vi "UHR-Fleezers Control (host) - 12.8.1.vi"() -> ()   [LabVIEW 2012] (continued)
          tunnel: [w4493 w4495] -> w4446
          tunnel: [w4492 w4494] -> w4445
          tunnel: w4448 -> [w4493 w4498]
          tunnel: w4447 -> [w4492 w4497]
          frame False {
          }
          frame True {
            n2536 = call "reset FPGA DMA.vi"("error in"=w4497, "FPGA VI Reference In"=w4498) -> ("error out"=w4494:errorcluster, "FPGA VI Reference Out"=w4495:T24)
            n2537 = local write "Overflow (data lost)"(FALSE ("Overflow (data lost)")) -> ()
          }
        }
        n2538 = case shown="False" w4436 {
          selector: w4436 -> [_ w4452]
          tunnel: w4435 -> [w4451 _]
          tunnel: [w4451 w4452] -> w4434
          frame False {
            n2539 = property on="2D or 1D Scan" class="Bool (strict)"("Val(Sgnl)"=w4451) -> ()  [unwired: 2 in, 2 out]
            n2540 = property on="Confocal Image" class="Bool (strict)"("Value"=FALSE ("Start Confocal Map")) -> ()  [unwired: 2 in, 2 out]
          }
          frame True {
          }
        }
        n2541 = local write "MCL Scanning"(w4441) -> ()
        n2542 = local read "AO1"() -> (w4438:dbl)
        n2543 = local read "AO2"() -> (w4437:dbl)
        n2544 = case shown="True" "Center Scan" {
          tunnel: w4446 -> [w4459 w4491]
          tunnel: w4445 -> [w4458 w4490]
          tunnel: [w4457 w4489] -> w4443
          tunnel: [w4456 w4488] -> w4442
          tunnel: [w4454 w4475] -> w4440
          tunnel: [w4453 w4474] -> w4439
          tunnel: w4438 -> [w4454 w4480]
          tunnel: w4437 -> [w4453 w4483]
          tunnel: w4434 -> [_ _]
          frame False {
            w4455 = TRUE ("AI to FIFO")
            n2545 = xnode "Read/Write Control"("FPGA VI Reference In"=w4459, "error in"=w4458, "AI to FIFO"=w4455, "APD to FIFO"=w4455, "Start scan (MCL)"=w4455) -> ("FPGA VI Reference Out"=w4457:T24, "error out"=w4456:errorcluster)
          }
          frame True {
            w4487 = TRUE ("AI to FIFO")
            n2546 = local read "Scan steps (MCL)"() -> (w4466:u64)
            n2547 = local read "Scan lines (y)"() -> (w4462:u64)
            n2548 = local read "Fast Scan Dir"() -> (w4473:bool)
            n2549 = local read "Actual MCL Inc (V)"() -> (w4463:dbl)
            n2550 = Decrement(x=w4462) -> (x-1=w4461:u64)
            n2551 = Decrement(x=w4466) -> (x-1=w4465:u64)
            n2552 = Multiply(x=w4463, y=w4461) -> (x*y=w4460:dbl)
            n2553 = Divide(x=w4460, y=2.0) -> (x/y=w4470:dbl)
            n2554 = Multiply(x=w4463, y=w4465) -> (x*y=w4464:dbl)
            n2555 = Divide(x=w4464, y=2.0) -> (x/y=w4469:dbl)
            n2556 = Select(t=w4469, s=w4473, f=w4470) -> (s? t:f=w4468:dbl)
            n2557 = Select(t=w4470, s=w4473, f=w4469) -> (s? t:f=w4472:dbl)
            n2558 = Subtract(x=w4480, y=w4472) -> (x-y=w4471:dbl)
            n2559 = Subtract(x=w4483, y=w4468) -> (x-y=w4467:dbl)
            n2560 = local read "2D or 1D Scan"() -> (w4485:bool)
            n2561 = Not(x=w4473) -> (.not. x?=w4479:bool)
            n2562 = Not(x=w4485) -> (.not. x?=w4481:bool)
            n2563 = And(x=w4473, y=w4481) -> (x .and. y?=w4482:bool)
            n2564 = And(x=w4481, y=w4479) -> (x .and. y?=w4484:bool)
            n2565 = Select(t=w4483, s=w4484, f=w4467) -> (s? t:f=w4474:dbl)
            n2566 = Select(t=w4480, s=w4482, f=w4471) -> (s? t:f=w4475:dbl)
            n2567 = call "Volt to I16.vi"("Voltage In"=w4475) -> ("I16 Voltage Out"=w4478:i16)
            n2568 = call "Volt to I16.vi"("Voltage In"=w4474) -> ("I16 Voltage Out"=w4477:i16)
            n2569 = xnode "Read/Write Control"("FPGA VI Reference In"=w4491, "error in"=w4490, "AI to FIFO"=w4487, "APD to FIFO"=w4487, "Start scan (MCL)"=w4487, "AO1"=w4478, "AO2"=w4477) -> ("FPGA VI Reference Out"=w4489:T24, "error out"=w4488:errorcluster)
          }
        }
        "Initial Y" <- w4440
        "Initial X" <- w4439
        n2570 = local write "Tab Control 6"(T3."Imaging" ("Tab Control 6")) -> ()
        "wait to reset values" <- w4441
      }
    }
    n2571 = local read "APD Elements/DMA read"() -> (w3617:u32)
    n2572 = local read "Trap AI Elements/DMA read"() -> (w3824:u32)
    n2573 = xnode "Get APD Data"("FPGA VI Reference In"=w3770, "error in"=w3769, "Number of Elements"=w3617, "Timeout (ms)"=-1) -> ("Data"=w3798:u32[], "Elements Remaining"=→"APD FIFO Elements Remaining":u32)  [unwired: 2 out]
    n2574 = local read "Trap Pos Elements/DMA read"() -> (w3766:u32)
    n2575 = xnode "Invoke Method"("FPGA VI Reference In"=w3770, "error in"=w3769, "Number of Elements"=w3766, "Timeout (ms)"=-1) -> ("Data"=w3730:u16[], "Elements Remaining"=→"Trap Pos FIFO El Remaining":u32)  [unwired: 2 out]
    n2576 = xnode "Get Trap Data"("FPGA VI Reference In"=w3770, "error in"=w3769, "Number of Elements"=w3824, "Timeout (ms)"=-1 ("Timeout")) -> ("FPGA VI Reference Out"=w3665:T24, "error out"=w3664:errorcluster, "Data"=w3731:i16[], "Elements Remaining"=w3923:u32)
    "FIFO El. Rem." <- w3923
    n2577 = local read "DMA Update Period (s)"() -> (w3825:dbl)
    n2578 = local read "Trap AI FIFO Depth"() -> (w3925:u32)
    n2579 = local read "Number of APDs"() -> (w3636:u8)
    n2580 = Decimate 1D Array(w3730) -> (w3727:u16[], w3729:u16[], w3728:u16[])
    n2581 = feedback #6(0.0) -> (w3759:dbl)
    n2582 = Add(x=w3825, y=w3759) -> (x+y=w3899:dbl)
    n2583 = feedback-in #6(w3899) -> ()
    n2584 = To Time Stamp(1:w3759) -> (0:w3758:timestamp)
    n2585 = Subtract(x=w3925, y=w3824) -> (x-y=w3924:u32)
    n2586 = To Unsigned Long Integer(number=w3727) -> (unsigned 32bit integer=w3726:u32[])
    n2587 = Join Numbers(hi=w3729, lo=w3728) -> ((hi.lo)=w3725:u32[])
    n2588 = Divide(x=w3923, y=w3924) -> (x/y=w3922:dbl)
    "Buffer Status" <- w3922
    n2589 = case "Deinterlace APD signals" shown="3, Default" w3636 {
      tunnel: [w3995 w4001] -> w3616
      tunnel: w3798 -> [w3996 w4000]
      tunnel: [w3994 w3999] -> w3615
      tunnel: [w3993 w3997] -> w3605
      frame 3, Default {
        n2590 = Decimate 1D Array "APD signals"(w3996) -> (w3995:u32[], w3994:u32[], w3993:u32[])
      }
      frame 2 {
        n2591 = Decimate 1D Array "APD signals"(w4000) -> (w4001:u32[], w3999:u32[])
        n2592 = Multiply(x=w3999, y=u32 0) -> (x*y=w3997:u32[])
      }
    }
    n2593 = Join Numbers(hi=w3726, lo=w3725) -> ((hi.lo)=w3719:u64[])
    n2594 = call "IR AOM word to freq - vec.vi"("Frequency Word In (double vec)"=w3719) -> ("Frequency Out"=w3765:dbl[])
    n2595 = Equal?(x=w3922, y=1.0) -> (x = y?=w3920:bool)
    n2596 = case "Alert buffer overflow" shown="True" w3920 {
      frame False {
      }
      frame True {
        n2597 = call <vilib>:"Beep.vi"() -> ()  [unwired: 3 in, 9 out]
        "Overflow (data lost)" <- TRUE ("Overflow (data lost)")
      }
    }
    n2598 = Decimate 1D Array(w3765) -> (w3764:dbl[], w3763:dbl[])
    n2599 = Build Array(w3764, w3763) -> (w3762:dbl[][])
    n2600 = Bundle(w3616, w3615, w3605) -> (w3620:cluster{u32[], u32[], u32[]})  [unwired: 1 in]
    n2601 = Build Array(w3616, w3615, w3605) -> (w3860:u32[][])
    n2602 = for {
      tunnel: w3616 -> [w3991] mode=indexing
      n2603 = call "Smart Buffer (DBL) 1.vi"("new element [write]"=w3991, "mode"=T25."write") -> ()  [unwired: 4 in, 6 out]
    }
    n2604 = local read "APD Integration Time (s)"() -> (w3631:dbl)
    n2605 = To Double Precision Float(number=w3860) -> (double precision float=w3861:dbl[][])
    n2606 = feedback #7 "APD3"(w3605) -> (w3606:u32[])
    n2607 = feedback #8 "APD2"(w3615) -> (w3788:u32[])
    n2608 = feedback #9 "APD1"(w3616) -> (w3859:u32[])
    n2609 = Build Array (concatenate)(w3788, w3615) -> (w3787:u32[])
    n2610 = Build Array (concatenate)(w3606, w3605) -> (w3604:u32[])
    n2611 = Build Array (concatenate)(w3859, w3616) -> (w3856:u32[])
    n2612 = for {
      tunnel: w3615 -> [w3990] mode=indexing
      n2613 = call "Smart Buffer (DBL) 2.vi"("new element [write]"=w3990, "mode"=T25."write") -> ()  [unwired: 4 in, 6 out]
    }
    n2614 = Array Size(array=w3856) -> (size(s)=w3853:i32)
    n2615 = Array Size(array=w3616) -> (size(s)=w3855:i32)
    n2616 = Multiply(x=w3855, y="APD Ave N") -> (x*y=w3854:dbl)
    n2617 = Greater?(x=w3853, y=w3854) -> (0:w3857:bool)
    n2618 = Bundle("APD 1", "APD 2", "APD 3") -> (w3893:cluster{string, string, string})  [unwired: 1 out]
    n2619 = local read "Trap Sets"() -> (w3823:u32)
    n2620 = case shown="True" w3857 {
      tunnel: w3856 -> [w4247 w4256]
      tunnel: [w4247 w4254] -> w3830
      tunnel: w3854 -> [_ w4249]
      tunnel: w3853 -> [_ w4255]
      tunnel: w3787 -> [w4246 w4253]
      tunnel: [w4246 w4252] -> w3785
      tunnel: w3604 -> [w4245 w4251]
      tunnel: [w4245 w4248] -> w3632
      frame False {
      }
      frame True {
        n2621 = Subtract(x=w4255, y=w4249) -> (x-y=w4250:dbl)
        n2622 = Array Subset "APD3"(array=w4251, index=w4250, length=w4249) -> (w4248:u32[])
        n2623 = Array Subset "APD2"(array=w4253, index=w4250, length=w4249) -> (w4252:u32[])
        n2624 = Array Subset "APD1"(array=w4256, index=w4250, length=w4249) -> (w4254:u32[])
      }
    }
    n2625 = feedback-in #7(w3632) -> ()
    n2626 = feedback-in #8(w3785) -> ()
    n2627 = feedback-in #9(w3830) -> ()
    n2628 = Cluster To Array(cluster=w3893) -> (array=w3890:string[])
    n2629 = for "APD" {
      tunnel: w3861 -> [w4503] mode=indexing
      tunnel: w3631 -> [w4510]
      tunnel: [w4506] -> w3789 mode=indexing
      tunnel: "APD Disp. Scale" -> [w4507]
      tunnel: w3890 -> [w4505] mode=indexing
      tunnel: "APD Disp. Downsample" -> [w4501]
      tunnel: [w4504] -> w3889
      workers-P: _ -> [_]
      tunnel: w3758 -> [w4500]
      n2630 = call "integrate 1D array interval - double.vi"("Ave N"=w4501, "Array In"=w4503) -> ("Array Out"=w4502:dbl[])  [unwired: 1 out]
      n2631 = Multiply(x=w4510, y=w4501) -> (x*y=w4504:dbl)
      n2632 = Divide(x=w4502, y=w4507) -> (x/y=w4508:dbl[])
      n2633 = Bundle By Name("t0"=w4500, "Y"=w4508, "dt"=w4504) -> (w4509:waveform(dbl))  [unwired: 1 out]
      n2634 = Set Waveform Attribute(5:w4505, 6:"NI_ChannelName" ("name"), 7:w4509) -> (3:w4506:waveform(dbl))  [unwired: 1 in, 2 out]
    }
    "APD Display Period (s)" <- w3889
    n2635 = Reciprocal(x=w3889) -> (1/x=→"APD Display Freq. (Hz)":dbl)
    n2636 = case "Deinterlace trap data, average down PSD" shown="2" w3823 {
      tunnel: w3731 -> [w4528 w4593]
      tunnel: [w4525 w4590] -> w3818
      tunnel: [w4528 w4592] -> w3722
      tunnel: "Detector Type" -> [w4527 w4588]
      tunnel: [w4526 w4591] -> w3817
      tunnel: [w4524 w4589] -> w3897
      frame 1, Default {
        n2637 = Divide(x=w4528, y=3276.7) -> (x/y=w4529:dbl[])
        n2638 = Decimate 1D Array(w4529) -> (w4538:dbl[], w4537:dbl[], w4536:dbl[], w4535:dbl[], w4534:dbl[], w4533:dbl[], w4532:dbl[], w4531:dbl[])
        n2639 = case shown="\"IR-QPD + PSD + FB-QPD position\"" w4527 {
          tunnel: w4538 -> [w4562 w4587]
          tunnel: w4537 -> [w4561 w4586]
          tunnel: w4536 -> [w4546 w4564]
          tunnel: w4535 -> [w4547 w4574]
          tunnel: w4534 -> [w4560 w4585]
          tunnel: w4533 -> [w4559 w4584]
          tunnel: w4532 -> [w4543 w4565]
          tunnel: w4531 -> [w4542 w4563]
          tunnel: [w4541 w4571] -> w4526
          tunnel: [w4540 w4570] -> w4525
          tunnel: [w4539 w4569] -> w4524
          frame "IR-QPD + PSD + FB-QPD", Default {
            w4539 = 0  # Channel pattern
            n2640 = Divide(x=w4562, y=w4547) -> (x/y=w4549:dbl[])
            n2641 = Divide(x=w4561, y=w4547) -> (x/y=w4548:dbl[])
            n2642 = Divide(x=w4560, y=w4543) -> (x/y=w4545:dbl[])
            n2643 = Divide(x=w4559, y=w4542) -> (x/y=w4544:dbl[])
            n2644 = Build Array(w4549, w4548, w4547, w4546, w4545, w4544, w4543, w4542) -> (w4540:dbl[][])
            n2645 = Bundle("T1 Y", "T1 X", "T1 Sum", "FB Sum", "PSD Y", "PSD X", "PSD Y Sum", "PSD X Sum") -> (w4558:T49)  [unwired: 1 out]
            n2646 = Cluster To Array(cluster=w4558) -> (array=w4541:string[])
          }
          frame "IR-QPD + PSD + FB-QPD position" {
            w4569 = 3  # Channel pattern
            n2647 = Negate(x=w4565) -> (-x=w4566:dbl[])
            n2648 = Divide(x=w4587, y=w4574) -> (x/y=w4576:dbl[])
            n2649 = Divide(x=w4586, y=w4574) -> (x/y=w4575:dbl[])
            n2650 = Divide(x=w4585, y=w4565) -> (x/y=w4573:dbl[])
            n2651 = Divide(x=w4584, y=w4566) -> (x/y=w4572:dbl[])
            n2652 = Build Array(w4576, w4575, w4574, w4563, w4564, w4573, w4572, w4565) -> (w4570:dbl[][])
            n2653 = Bundle("T1 Y", "T1 X", "T1 Sum", "FB X", "FB Sum", "PSD Y", "PSD X", "PSD Y Sum") -> (w4583:T49)  [unwired: 1 out]
            n2654 = Cluster To Array(cluster=w4583) -> (array=w4571:string[])
          }
        }
      }
      frame 2 {
        n2655 = case shown="\"IR-QPD + PSD + FB-QPD X position\", Default" w4588 {
          tunnel: w4593 -> [w4655 w4727 w4798]
          tunnel: [w4594 w4718 w4729] -> w4592
          tunnel: [w4621 w4709 w4776] -> w4591
          tunnel: [w4620 w4672 w4743] -> w4590
          tunnel: [w4614 w4707 w4774] -> w4589
          frame "IR-QPD + PSD + FB-QPD" {
            w4614 = 1  # Channel pattern
            # "time average x2 the 4th signal and the 4 psd signals (detection laser)"
            # "deinterlace 3 signals from qpd"
            n2656 = Decimate 1D Array(w4655) -> (w4654:i16[], w4653:i16[], w4619:i16[], w4652:i16[], w4642:i16[], w4640:i16[], w4639:i16[], w4637:i16[])
            n2657 = Decimate 1D Array(w4619) -> (w4618:i16[], w4617:i16[])
            n2658 = Decimate 1D Array(w4654) -> (w4651:i16[], w4623:i16[])
            n2659 = Decimate 1D Array(w4653) -> (w4650:i16[], w4648:i16[])
            n2660 = Decimate 1D Array(w4652) -> (w4649:i16[], w4647:i16[])
            n2661 = call "downsample 1D array - double.vi"("Ave N"=2.0, "Array In"=w4642) -> ("Array Out"=w4641:dbl[])  [unwired: 1 out]
            n2662 = call "downsample 1D array - double.vi"("Ave N"=2.0, "Array In"=w4640) -> ("Array Out"=w4622:dbl[])  [unwired: 1 out]
            n2663 = call "downsample 1D array - double.vi"("Ave N"=2.0, "Array In"=w4639) -> ("Array Out"=w4638:dbl[])  [unwired: 1 out]
            n2664 = call "downsample 1D array - double.vi"("Ave N"=2.0, "Array In"=w4637) -> ("Array Out"=w4636:dbl[])  [unwired: 1 out]
            n2665 = Interleave 1D Arrays(w4651, w4650, w4649, w4623, w4648, w4647, w4618, w4617, w4641, w4622, w4638, w4636) -> (w4635:dbl[])
            n2666 = Divide(x=w4635, y=3276.7) -> (x/y=w4634:dbl[])
            n2667 = Decimate 1D Array(w4634) -> (w4633:dbl[], w4632:dbl[], w4631:dbl[], w4630:dbl[], w4629:dbl[], w4628:dbl[], w4616:dbl[], w4615:dbl[], w4627:dbl[], w4626:dbl[], w4625:dbl[], w4624:dbl[])
            n2668 = Divide(x=w4633, y=w4631) -> (x/y=w4601:dbl[])
            n2669 = Divide(x=w4632, y=w4631) -> (x/y=w4600:dbl[])
            n2670 = Divide(x=w4630, y=w4628) -> (x/y=w4599:dbl[])
            n2671 = Divide(x=w4629, y=w4628) -> (x/y=w4598:dbl[])
            n2672 = Divide(x=w4627, y=w4625) -> (x/y=w4597:dbl[])
            n2673 = Divide(x=w4626, y=w4624) -> (x/y=w4596:dbl[])
            n2674 = Build Array(w4601, w4600, w4631, w4599, w4598, w4628, w4616, w4615, w4597, w4596, w4625, w4624) -> (w4620:dbl[][])
            n2675 = Bundle("T1 Y", "T1 X", "T1 Sum", "T2 Y", "T2 X", "T2 Sum", "T1 FB Sum", "T2 FB Sum", "PSD Y", "PSD X", "PSD Y Sum", "PSD X Sum") -> (w4602:T50)  [unwired: 1 out]
            n2676 = To Word Integer(number=w4635) -> (16bit integer=w4594:i16[])
            n2677 = Cluster To Array(cluster=w4602) -> (array=w4621:string[])
          }
          frame "IR-QPD + PSD + FB-QPD X position", Default {
            w4707 = 2  # Channel pattern
            # "time average x2 the 3 psd signals (detection laser)"
            # "deinterlace 3 signals from qpds"
            n2678 = Decimate 1D Array(w4727) -> (w4726:i16[], w4725:i16[], w4708:i16[], w4724:i16[], w4670:i16[], w4667:i16[], w4664:i16[], w4695:i16[])
            n2679 = Select(t=i16 -1, s="Flip X Sign", f=i16 1) -> (s? t:f=w4660:i16)
            n2680 = Multiply(x=w4725, y=w4660) -> (x*y=w4661:i16[])
            n2681 = Decimate 1D Array(w4708) -> (w4693:i16[], w4691:i16[])
            n2682 = Decimate 1D Array(w4726) -> (w4723:i16[], w4710:i16[])
            n2683 = Decimate 1D Array(w4661) -> (w4722:i16[], w4720:i16[])
            n2684 = Decimate 1D Array(w4724) -> (w4721:i16[], w4719:i16[])
            n2685 = Decimate 1D Array(w4695) -> (w4694:i16[], w4692:i16[])
            n2686 = call "downsample 1D array - I16.vi"("Ave N"=2.0, "Array In"=w4670) -> ("Array Out"=w4668:i16[])  [unwired: 1 in]
            n2687 = call "downsample 1D array - I16.vi"("Ave N"=2.0, "Array In"=w4664) -> ("Array Out"=w4662:i16[])  [unwired: 1 in]
            n2688 = call "downsample 1D array - I16.vi"("Ave N"=2.0, "Array In"=w4667) -> ("Array Out"=w4665:i16[])  [unwired: 1 in]
            n2689 = Interleave 1D Arrays(w4723, w4722, w4721, w4710, w4720, w4719, w4694, w4693, w4692, w4691, w4668, w4665, w4662) -> (w4718:i16[])
            n2690 = Divide(x=w4718, y=3276.7) -> (x/y=w4717:dbl[])
            n2691 = Decimate 1D Array(w4717) -> (w4716:dbl[], w4715:dbl[], w4714:dbl[], w4713:dbl[], w4712:dbl[], w4711:dbl[], w4683:dbl[], w4681:dbl[], w4680:dbl[], w4678:dbl[], w4677:dbl[], w4676:dbl[], w4673:dbl[])
            n2692 = Negate(x=w4673) -> (-x=w4671:dbl[])
            n2693 = Divide(x=w4677, y=w4673) -> (x/y=w4675:dbl[])
            n2694 = Divide(x=w4676, y=w4671) -> (x/y=w4674:dbl[])
            n2695 = Divide(x=w4716, y=w4714) -> (x/y=w4699:dbl[])
            n2696 = Divide(x=w4715, y=w4714) -> (x/y=w4698:dbl[])
            n2697 = Divide(x=w4713, y=w4711) -> (x/y=w4697:dbl[])
            n2698 = Divide(x=w4712, y=w4711) -> (x/y=w4696:dbl[])
            n2699 = Divide(x=w4683, y=w4681) -> (x/y=w4682:dbl[])
            n2700 = Divide(x=w4680, y=w4678) -> (x/y=w4679:dbl[])
            n2701 = Build Array(w4699, w4698, w4714, w4697, w4696, w4711, w4682, w4681, w4679, w4678, w4675, w4674, w4673) -> (w4672:dbl[][])
            n2702 = Bundle("T1 Y", "T1 X", "T1 Sum", "T2 Y", "T2 X", "T2 Sum", "T1 FB X", "T1 FB Sum", "T2 FB X", "T2 FB Sum", "PSD Y", "PSD X", "PSD Y Sum") -> (w4700:T51)  [unwired: 1 out]
            n2703 = Cluster To Array(cluster=w4700) -> (array=w4709:string[])
          }
          frame "IR-QPD + PSD + FB-QPD XY positions" {
            w4774 = 4  # Channel pattern
            # "time average x2 the 3 psd signals (detection laser)"
            # "deinterlace 3 signals from qpds"
            n2704 = Decimate 1D Array(w4798) -> (w4797:i16[], w4796:i16[], w4775:i16[], w4795:i16[], w4741:i16[], w4787:i16[], w4786:i16[], w4763:i16[])
            n2705 = Decimate 1D Array "Feedback Sum"(w4775) -> (w4759:i16[], w4757:i16[])
            n2706 = Decimate 1D Array "QPD Y"(w4797) -> (w4794:i16[], w4777:i16[])
            n2707 = Decimate 1D Array "QPD X"(w4796) -> (w4793:i16[], w4791:i16[])
            n2708 = Decimate 1D Array "Feedback Y"(w4741) -> (w4740:i16[], w4739:i16[])
            n2709 = Decimate 1D Array "QPD Sum"(w4795) -> (w4792:i16[], w4790:i16[])
            n2710 = Decimate 1D Array "Feedback X"(w4763) -> (w4760:i16[], w4758:i16[])
            n2711 = call "downsample 1D array - double.vi"("Ave N"=2.0, "Array In"=w4787) -> ("Array Out"=w4762:dbl[])  [unwired: 1 out]
            n2712 = call "downsample 1D array - double.vi"("Ave N"=2.0, "Array In"=w4786) -> ("Array Out"=w4761:dbl[])  [unwired: 1 out]
            n2713 = Interleave 1D Arrays(w4794, w4793, w4792, w4777, w4791, w4790, w4740, w4760, w4759, w4739, w4758, w4757, w4762, w4761) -> (w4785:dbl[])
            n2714 = Divide(x=w4785, y=3276.7) -> (x/y=w4784:dbl[])
            n2715 = Decimate 1D Array(w4784) -> (w4783:dbl[], w4782:dbl[], w4781:dbl[], w4780:dbl[], w4779:dbl[], w4778:dbl[], w4736:dbl[], w4750:dbl[], w4734:dbl[], w4735:dbl[], w4748:dbl[], w4732:dbl[], w4746:dbl[], w4744:dbl[])
            n2716 = Negate(x=w4744) -> (-x=w4742:dbl[])
            n2717 = Divide(x=w4746, y=w4742) -> (x/y=w4745:dbl[])
            n2718 = Divide(x=w4735, y=w4732) -> (x/y=w4731:dbl[])
            n2719 = Divide(x=w4736, y=w4734) -> (x/y=w4733:dbl[])
            n2720 = Divide(x=w4783, y=w4781) -> (x/y=w4767:dbl[])
            n2721 = Divide(x=w4782, y=w4781) -> (x/y=w4766:dbl[])
            n2722 = Divide(x=w4780, y=w4778) -> (x/y=w4765:dbl[])
            n2723 = Divide(x=w4779, y=w4778) -> (x/y=w4764:dbl[])
            n2724 = Divide(x=w4750, y=w4734) -> (x/y=w4749:dbl[])
            n2725 = Divide(x=w4748, y=w4732) -> (x/y=w4747:dbl[])
            n2726 = Build Array(w4767, w4766, w4781, w4765, w4764, w4778, w4733, w4749, w4734, w4731, w4747, w4732, w4745, w4744) -> (w4743:dbl[][])
            n2727 = Bundle("T1 Y", "T1 X", "T1 Sum", "T2 Y", "T2 X", "T2 Sum", "T1 FB Y", "T1 FB X", "T1 FB Sum", "T2 FB Y", "T2 FB X", "T2 FB Sum", "PSD X", "PSD Y Sum") -> (w4730:T52)  [unwired: 1 out]
            n2728 = To Word Integer(number=w4785) -> (16bit integer=w4729:i16[])
            n2729 = Cluster To Array(cluster=w4730) -> (array=w4776:string[])
          }
        }
      }
    }
    "AI labels" <- w3817
    n2730 = local read "APD Integration Time (s)"() -> (w3794:dbl)
    n2731 = Array Size(array=w3830) -> (size(s)=w3852:i32)
    n2732 = call <vilib>:"Std Deviation and Variance.vi"("X"=w3785) -> ("standard deviation"=w3784:dbl)  [unwired: 1 in, 2 out]
    n2733 = Add Array Elements(numeric array=w3785) -> (sum=w3786:u32)
    n2734 = Add Array Elements(numeric array=w3830) -> (sum=w3862:u32)
    n2735 = call <vilib>:"Std Deviation and Variance.vi"("X"=w3830) -> ("standard deviation"=w3829:dbl)  [unwired: 1 in, 2 out]
    n2736 = Divide(x=w3784, y=w3631) -> (x/y=w3781:dbl)
    "Rate sigma (Hz) 2" <- w3781
    n2737 = Multiply(x=w3631, y=w3852) -> (x*y=w3633:dbl)
    "Int. Time (s)" <- w3633
    n2738 = Divide(x=w3786, y=w3633) -> (x/y=w3782:dbl)
    "APD 2 Rate (Hz)" <- w3782
    n2739 = Multiply(x="APD Disp. Scale", y=w3789) -> (x*y=w3796:waveform(dbl)[])
    n2740 = Divide(x=w3862, y=w3633) -> (x/y=w3827:dbl)
    "APD 1 Rate (Hz)" <- w3827
    n2741 = Divide(x=w3829, y=w3631) -> (x/y=w3828:dbl)
    "Rate sigma (Hz)" <- w3828
    n2742 = Divide(x=w3781, y=w3782) -> (x/y=→"Sigma/Mean 2":dbl)
    n2743 = Multiply(x="APD Disp. Downsample", y=w3794) -> (x*y=w3792:dbl)
    n2744 = Divide(x=w3828, y=w3827) -> (x/y=→"Sigma/Mean":dbl)
    n2745 = Divide(x=w3796, y=w3792) -> (x/y=w3623:waveform(dbl)[])
    n2746 = Index Array(array=w3623, index=0) -> (element=w3778:waveform(dbl))
    n2747 = Index Array(array=w3623, index=1) -> (element=w3776:waveform(dbl))
    n2748 = Index Array(array=w3623, index=2) -> (element=w3625:waveform(dbl))
    n2749 = Subtract(x=w3778, y="APD 1 Offset") -> (x-y=w3774:waveform(dbl))
    n2750 = Subtract(x=w3776, y="APD 2 Offset") -> (x-y=w3773:waveform(dbl))
    n2751 = Subtract(x=w3625, y="APD 3 Offset") -> (x-y=w3622:waveform(dbl))
    n2752 = Add Array Elements(numeric array=w3632) -> (sum=w3635:u32)
    n2753 = call <vilib>:"Std Deviation and Variance.vi"("X"=w3632) -> ("standard deviation"=w3634:dbl)  [unwired: 1 in, 2 out]
    n2754 = Build Array(w3774, w3773, w3622) -> (→"APD Chart":waveform(dbl)[])
    n2755 = Divide(x=w3635, y=w3633) -> (x/y=w3629:dbl)
    "APD 3 Rate (Hz)" <- w3629
    n2756 = Divide(x=w3634, y=w3631) -> (x/y=w3630:dbl)
    "Rate sigma (Hz) 3" <- w3630
    n2757 = Divide(x=w3630, y=w3629) -> (x/y=→"Sigma/Mean 3":dbl)
    n2758 = local read "Data Period (s)"() -> (w3681:dbl)
    n2759 = local read "BD 1 Frequency 2 (MHz)"() -> (w3714:dbl)
    n2760 = local read "BD 1 Frequency 1 (MHz)"() -> (w3715:dbl)
    n2761 = Decimate 1D Array(w3722) -> (w3746:i16[], w3745:i16[], w3743:i16[], w3742:i16[])  [unwired: 9 out]
    n2762 = Multiply(x=w3681, y="Trap Pos. Disp. Downsample") -> (x*y=w3679:dbl)
    n2763 = Divide(x=w3746, y=w3745) -> (x/y=w3747:dbl[])
    n2764 = Divide(x=w3743, y=w3742) -> (x/y=w3744:dbl[])
    n2765 = local read "AOM X Cal (nm/MHz)"() -> (w3712:dbl)
    n2766 = Split 1D Array(array=w3747, index="N El. to Ave.") -> (second subarray=w3750:dbl[])  [unwired: 1 out]
    n2767 = Split 1D Array(array=w3744, index="N El. to Ave.") -> (second subarray=w3749:dbl[])  [unwired: 1 out]
    n2768 = Multiply(x=w3681, y="Trap Disp. Downsample") -> (x*y=w3760:dbl)
    "Display Period (s)" <- w3760
    n2769 = for "Trap AI" {
      tunnel: [w4523] -> w3584 mode=indexing
      tunnel: w3758 -> [w4514]
      tunnel: "Trap Disp. Downsample" -> [w4521]
      tunnel: w3818 -> [w4519] mode=indexing
      tunnel: w3681 -> [w4518]
      tunnel: w3817 -> [w4517] mode=indexing
      tunnel: [w4516] -> w3791 mode=indexing
      tunnel: w3760 -> [w4515]
      workers-P: _ -> [_]
      n2770 = Bundle By Name("Y"=w4519, "dt"=w4518) -> (w4520:waveform(dbl))  [unwired: 1 out]
      n2771 = Set Waveform Attribute(5:w4517, 6:"NI_ChannelName" ("name"), 7:w4520) -> (3:w4516:waveform(dbl))  [unwired: 1 in, 2 out]
      n2772 = call "downsample 1D array - double.vi"("Ave N"=w4521, "Array In"=w4519) -> ("Array Out"=w4522:dbl[])  [unwired: 1 out]
      n2773 = Bundle By Name(cluster=w4516, "t0"=w4514, "Y"=w4522, "dt"=w4515) -> (w4523:waveform(dbl))
    }
    n2774 = Bundle("BD 1 Frequency 1 (MHz)"=w3715, "BD 1 Frequency 2 (MHz)"=w3714) -> (w3716:T53)  [unwired: 1 out]
    n2775 = call-poly <vilib>:"Mean.vi"("X"=w3749) -> ("mean"=w3737:dbl)  [unwired: 1 out]
    n2776 = call-poly <vilib>:"Mean.vi"("X"=w3750) -> ("mean"=w3738:dbl)  [unwired: 1 out]
    n2777 = Reciprocal(x=w3760) -> (1/x=→"Trap Disp. Freq. (Hz)":dbl)
    n2778 = Cluster To Array(cluster=w3716) -> (array=w3713:dbl[])
    n2779 = local read "Trap X AI1 (DMA)"() -> (w3748:T15)
    n2780 = local read "Data points/scans (MCL)"() -> (w3872:dbl)
    n2781 = To Fixed-Point(number=w3737) -> (fixed-point=w3735:fxp<+/-,16,1>)  [unwired: 1 in]
    n2782 = To Fixed-Point(number=w3738) -> (fixed-point=w3736:fxp<+/-,16,1>)  [unwired: 1 in]
    n2783 = Bundle("Trap 1 Pos.", "Trap 2 Pos.") -> (w3757:cluster{string, string})  [unwired: 1 out]
    n2784 = Bundle By Name(cluster=w3748, "Set 1"=w3736, "Set 2"=w3735) -> (→"Trap X AI1 (DMA)":T15)
    n2785 = Cluster To Array(cluster=w3757) -> (array=w3754:string[])
    n2786 = Unbundle(w3620) -> (w3621:u32[])  [unwired: 2 out]
    n2787 = Select(t=-1.0, s="Negate Y Axis", f=1.0) -> (s? t:f=w3698:dbl)
    n2788 = for "Trap Position" {
      tunnel: w3762 -> [w4161] mode=indexing
      tunnel: "Trap Pos. Disp. Downsample" -> [w4160]
      tunnel: w3679 -> [w4158]
      tunnel: w3758 -> [w4157]
      tunnel: w3754 -> [w4155] mode=indexing
      tunnel: [w4154] -> w3668 mode=indexing
      tunnel: w3713 -> [w4152] mode=indexing
      tunnel: w3712 -> [w4150]
      tunnel: w3698 -> [w4149]
      n2789 = call "downsample 1D array - double.vi"("Ave N"=w4160, "Array In"=w4161) -> ("Array Out"=w4159:dbl[])  [unwired: 1 out]
      n2790 = Subtract(x=w4159, y=w4152) -> (x-y=w4153:dbl[])
      n2791 = Multiply(x=w4150, y=w4153) -> (x*y=w4151:dbl[])
      n2792 = Multiply(x=w4149, y=w4151) -> (x*y=w4148:dbl[])
      n2793 = Bundle By Name("Y"=w4148, "dt"=w4158, "t0"=w4157) -> (w4156:waveform(dbl))  [unwired: 1 out]
      n2794 = Set Waveform Attribute(5:w4155, 6:"NI_ChannelName" ("name"), 7:w4156) -> (3:w4154:waveform(dbl))  [unwired: 1 in, 2 out]
    }
    n2795 = To Double Precision Float(number=w3621) -> (double precision float=w3815:dbl[])
    n2796 = local read "Display Period (s)"() -> (w3806:dbl)
    n2797 = Increment(x=w3872) -> (x+1=w3873:dbl)
    n2798 = Index Array(array=w3668, index=0) -> (element=w3672:waveform(dbl))
    n2799 = Index Array(array=w3668, index=1) -> (element=w3667:waveform(dbl))
    n2800 = feedback #10(w3873) -> (w3876:dbl)
    n2801 = Select(t=0, s=w3863, f=w3876) -> (s? t:f=w3869:dbl)
    n2802 = Array Size(array=w3815) -> (size(s)=w3875:i32)
    n2803 = Add(x=w3875, y=w3869) -> (x+y=w3870:dbl)
    n2804 = Unbundle By Name(w3672) -> ("Y"=w3673:dbl[])
    n2805 = Divide(x="Bead Sep. Int. Time (s)", y=w3806) -> (x/y=w3708:dbl)
    n2806 = Add(x=w3673, y="FB Trap Pos Offset") -> (x+y=w3671:dbl[])
    "T1 x pos data" <- w3671
    n2807 = Greater?(x=w3870, y=w3872) -> (0:w3871:bool)
    n2808 = feedback #11(w3671) -> (w3710:dbl[])
    n2809 = Build Array (concatenate)(w3671, w3710) -> (w3709:dbl[])
    n2810 = Bundle By Name(cluster=w3672, "Y"=w3671) -> (w3670:waveform(dbl))
    n2811 = Select(t=w3869, s=w3871, f=w3870) -> (s? t:f=w3868:dbl)
    n2812 = feedback-in #10(w3868) -> ()
    n2813 = local read "MCL Scanning"() -> (w3866:bool)
    n2814 = Bundle(w3670, w3667) -> (w3666:cluster{waveform(dbl), waveform(dbl)})  [unwired: 1 out]
    n2815 = Index Array(array=w3584, index="index 1") -> (element=w3610:waveform(dbl))
    n2816 = Index Array(array=w3584, index="index 2") -> (element=w3614:waveform(dbl))
    n2817 = Split 1D Array(array=w3709, index=w3708) -> (first subarray=w3702:dbl[])  [unwired: 1 out]
    n2818 = feedback-in #11(w3702) -> ()
    n2819 = Unbundle By Name(w3610) -> ("Y"=w3609:dbl[])
    n2820 = Unbundle By Name(w3614) -> ("Y"=w3613:dbl[])
    n2821 = Not(x=w3871) -> (.not. x?=w3865:bool)
    n2822 = Cluster To Array(cluster=w3666) -> (array=w3645:waveform(dbl)[])
    "Trap Positions" <- w3645
    n2823 = call-poly <vilib>:"Mean.vi"("X"=w3702) -> ("mean"=w3701:dbl)  [unwired: 1 out]
    "Mean T1 Position (nm)" <- w3701
    n2824 = Subtract(x=w3702, y=w3701) -> (x-y=w3707:dbl[])
    n2825 = Square(x=w3707) -> (x^2=w3706:dbl[])
    n2826 = And(x=w3865, y=w3866) -> (x .and. y?=w3867:bool)
    n2827 = call-poly <vilib>:"Mean.vi"("X"=w3706) -> ("mean"=w3705:dbl)  [unwired: 1 out]
    n2828 = call-poly <vilib>:"Mean.vi"("X"=w3609) -> ("mean"=→"Trap 1 sum mean":dbl)  [unwired: 1 out]
    n2829 = call-poly <vilib>:"Mean.vi"("X"=w3613) -> ("mean"=→"Trap 2 sum mean":dbl)  [unwired: 1 out]
    n2830 = Square Root(x=w3705) -> (sqrt(x)=w3704:dbl)
    n2831 = Or(x=w3867, y=w3863) -> (x .or. y?=w3864:bool)
    n2832 = Build Array (concatenate)(w3789, w3584) -> (→"All Signals":waveform(dbl)[])
    n2833 = Equal?(x="Tab Control 6", y=T43."High Res Display") -> (x = y?=w3819:bool)
    n2834 = case shown="False" "X or Y?" {
      tunnel: w3584 -> [w3980 w3986]
      tunnel: [w3981 w3985] -> w3579
      tunnel: [w3979 w3984] -> w3576
      frame False {
        n2835 = Index Array(array=w3980, index=0) -> (element=w3981:waveform(dbl))
        n2836 = Index Array(array=w3980, index=3) -> (element=w3979:waveform(dbl))
      }
      frame True {
        n2837 = Index Array(array=w3986, index=1) -> (element=w3985:waveform(dbl))
        n2838 = Index Array(array=w3986, index=4) -> (element=w3984:waveform(dbl))
      }
    }
    n2839 = Multiply(x=10.0, y=w3704) -> (x*y=→"Trap 1 Position RMS (A)":dbl)
    n2840 = case "For displaying the high resolution display (no downsampling)" shown="True" w3819 {
      tunnel: w3791 -> [_ w4181]
      frame False {
      }
      frame True {
        n2841 = Index Array(array=w4181, index="High Res. Display") -> (element=w4182:waveform(dbl))
        n2842 = call <vilib>:"Std Deviation and Variance.vi"("X"=w4182) -> ("mean"=w4189:dbl, "standard deviation"=w4194:dbl)  [unwired: 1 in, 1 out]
        "Mean Intensity" <- w4189
        "Sigma" <- w4194
        n2843 = Subtract(x=w4182, y=w4189) -> (x-y=w4188:waveform(dbl))
        n2844 = Select(t=w4188, s="Subtract mean", f=w4182) -> (s? t:f=→"1 Channel":waveform(dbl))
        n2845 = Divide(x=w4194, y=w4189) -> (x/y=→"Sigma/Mean":dbl)
        n2846 = feedback #12(1) -> (w4183:i32)
        n2847 = Greater Or Equal?(x=w4183, y="Slow mean N ave.") -> (x >= y?=w4196:bool)
        n2848 = Increment(x=w4183) -> (x+1=w4198:i32)
        n2849 = Select(t=1, s=w4196, f=w4198) -> (s? t:f=w4185:i32)
        n2850 = feedback-in #12(w4185) -> ()
        n2851 = feedback #13() -> (w4186:waveform(dbl))  [unwired: 1 out]
        n2852 = case shown="Default" w4183 {
          tunnel: [w4201 w4204] -> w4187
          tunnel: w4186 -> [w4203 _]
          tunnel: w4182 -> [w4202 w4204]
          frame Default {
            n2853 = call-poly <vilib>:"Append Waveforms.vi"("waveform B"=w4202, "waveform A"=w4203) -> ("waveform out"=w4201:waveform(dbl))  [unwired: 1 in, 8 out]
          }
          frame 1 {
          }
        }
        n2854 = feedback-in #13(w4187) -> ()
        n2855 = case shown="True" w4196 {
          tunnel: w4187 -> [_ w4200]
          frame False {
          }
          frame True {
            n2856 = call-poly <vilib>:"Mean.vi"("X"=w4200) -> ("mean"=→"Slow mean":dbl)  [unwired: 1 out]
          }
        }
      }
    }
    n2857 = case "For plotting results of scanning MCL (fluorescence and detection laser images)" shown="True" w3864 {
      tunnel: w3863 -> [_ w4264]
      tunnel: w3872 -> [_ _]
      tunnel: w3791 -> [_ w4391]
      tunnel: w3771 -> [_ w4299]
      tunnel: w3620 -> [_ w4270]
      frame False {
      }
      frame True {
        w4280 = u32 0 items=["Horizontal", "Vertical", "Central", "1st Diagonal", "2nd Diagonal"] ("Type of Symmetry")
        w4306 = u32 0 items=["Horizontal", "Vertical", "Central", "1st Diagonal", "2nd Diagonal"] ("Type of Symmetry")
        w4330 = u32 0 items=["Horizontal", "Vertical", "Central", "1st Diagonal", "2nd Diagonal"] ("Type of Symmetry")
        w4333 = u32 0 items=["Horizontal", "Vertical", "Central", "1st Diagonal", "2nd Diagonal"] ("Type of Symmetry")
        w4362 = u32 0 items=["Horizontal", "Vertical", "Central", "1st Diagonal", "2nd Diagonal"] ("Type of Symmetry")
        n2858 = Unbundle(w4270) -> (w4269:u32[], w4267:u32[], w4265:u32[])
        n2859 = To Double Precision Float(number=w4269) -> (double precision float=w4268:dbl[])
        n2860 = To Double Precision Float(number=w4267) -> (double precision float=w4266:dbl[])
        n2861 = To Double Precision Float(number=w4265) -> (double precision float=w4258:dbl[])
        n2862 = Index Array(array=w4391, index=10) -> (element=w4397:waveform(dbl))
        n2863 = Index Array(array=w4391, index=11) -> (element=w4394:waveform(dbl))
        n2864 = local read "Cycles/step (MCL)"() -> (w4347:u64)
        n2865 = Index Array(array=w4391, index="Channel") -> (element=w4393:waveform(dbl))
        n2866 = Unbundle(w4299) -> ("New Image"=w4298:T2, "New Image"=w4297:T2, "New Image"=w4271:T2, "New Image"=w4272:T2, "New Image"=w4273:T2)
        n2867 = local read "Scan steps (MCL)"() -> (w4260:u64)
        n2868 = Unbundle By Name(w4397) -> ("Y"=w4349:dbl[])
        n2869 = Unbundle By Name(w4394) -> ("Y"=w4351:dbl[])
        n2870 = local read "Scan lines (y)"() -> (w4261:u64)
        n2871 = local read "N APD Samp/step"() -> (w4263:dbl)
        n2872 = Unbundle By Name(w4393) -> ("Y"=w4356:dbl[])
        n2873 = call "downsample 1D array - double.vi"("Ave N"=w4347, "Array In"=w4349) -> ("Array Out"=w4348:dbl[])  [unwired: 1 out]
        n2874 = call "downsample 1D array - double.vi"("Ave N"=w4347, "Array In"=w4351) -> ("Array Out"=w4350:dbl[])  [unwired: 1 out]
        n2875 = call "downsample 1D array - double.vi"("Ave N"=w4347, "Array In"=w4356) -> ("Array Out"=w4355:dbl[])  [unwired: 1 out]
        n2876 = Multiply(x=w4260, y=u64 2) -> (x*y=w4262:u64)
        n2877 = feedback #14(w4266) -> (w4324:dbl[])
        n2878 = Build Array (concatenate)(w4324, w4266) -> (w4323:dbl[])
        n2879 = feedback #15(w4258) -> (w4259:dbl[])
        n2880 = Build Array (concatenate)(w4259, w4258) -> (w4257:dbl[])
        n2881 = Select(t=w4266, s=w4264, f=w4323) -> (s? t:f=w4308:dbl[])
        n2882 = feedback-in #14(w4308) -> ()
        n2883 = Select(t=w4258, s=w4264, f=w4257) -> (s? t:f=w4282:dbl[])
        n2884 = feedback-in #15(w4282) -> ()
        n2885 = feedback #16(w4268) -> (w4417:dbl[])
        n2886 = Build Array (concatenate)(w4417, w4268) -> (w4399:dbl[])
        n2887 = Select(t=w4268, s=w4264, f=w4399) -> (s? t:f=w4403:dbl[])
        n2888 = feedback-in #16(w4403) -> ()
        n2889 = feedback #17(w4348) -> (w4405:dbl[])
        n2890 = Build Array (concatenate)(w4405, w4348) -> (w4396:dbl[])
        n2891 = feedback #18(w4355) -> (w4415:dbl[])
        n2892 = Build Array (concatenate)(w4415, w4355) -> (w4414:dbl[])
        n2893 = feedback #19(w4350) -> (w4407:dbl[])
        n2894 = Build Array (concatenate)(w4407, w4350) -> (w4408:dbl[])
        n2895 = Select(t=w4348, s=w4264, f=w4396) -> (s? t:f=w4352:dbl[])
        n2896 = feedback-in #17(w4352) -> ()
        n2897 = Select(t=w4355, s=w4264, f=w4414) -> (s? t:f=w4354:dbl[])
        n2898 = feedback-in #18(w4354) -> ()
        n2899 = Select(t=w4350, s=w4264, f=w4408) -> (s? t:f=w4353:dbl[])
        n2900 = feedback-in #19(w4353) -> ()
        n2901 = call "integrate 1D array interval - double.vi"("Ave N"=w4263, "Array In"=w4308) -> ("Array Out"=w4319:dbl[])  [unwired: 1 out]
        n2902 = call "integrate 1D array interval - double.vi"("Ave N"=w4263, "Array In"=w4282) -> ("Array Out"=w4293:dbl[])  [unwired: 1 out]
        n2903 = call "integrate 1D array interval - double.vi"("Ave N"=w4263, "Array In"=w4403) -> ("Array Out"=w4402:dbl[])  [unwired: 1 out]
        n2904 = Array Size(array=w4319) -> (size(s)=w4320:i32)
        n2905 = Array Size(array=w4293) -> (size(s)=w4294:i32)
        n2906 = Array Size(array=w4402) -> (size(s)=w4404:i32)
        n2907 = Multiply(x=w4261, y=w4262) -> (x*y=w4322:u64)
        n2908 = Multiply(x=w4261, y=w4262) -> (x*y=w4296:u64)
        n2909 = Multiply(x=w4261, y=w4262) -> (x*y=w4412:u64)
        n2910 = Subtract(x=w4322, y=w4320) -> (x-y=w4313:u64)
        n2911 = call-poly <vilib>:"Mean.vi"("X"=w4319) -> ("mean"=w4310:dbl)  [unwired: 1 out]
        n2912 = Subtract(x=w4296, y=w4294) -> (x-y=w4287:u64)
        n2913 = call-poly <vilib>:"Mean.vi"("X"=w4293) -> ("mean"=w4284:dbl)  [unwired: 1 out]
        n2914 = Subtract(x=w4412, y=w4404) -> (x-y=w4346:u64)
        n2915 = call-poly <vilib>:"Mean.vi"("X"=w4402) -> ("mean"=w4343:dbl)  [unwired: 1 out]
        n2916 = call-poly <vilib>:"Mean.vi"("X"=w4352) -> ("mean"=w4336:dbl)  [unwired: 1 out]
        n2917 = call-poly <vilib>:"Mean.vi"("X"=w4354) -> ("mean"=w4341:dbl)  [unwired: 1 out]
        n2918 = call-poly <vilib>:"Mean.vi"("X"=w4353) -> ("mean"=w4339:dbl)  [unwired: 1 out]
        n2919 = Initialize Array(1.0 ("element"), w4313) -> (w4309:dbl[])
        n2920 = Initialize Array(1.0 ("element"), w4287) -> (w4283:dbl[])
        n2921 = Initialize Array(1.0 ("element"), w4346) -> (w4337:dbl[])
        n2922 = Multiply(x=w4309, y=w4310) -> (x*y=w4311:dbl[])
        n2923 = Multiply(x=w4283, y=w4284) -> (x*y=w4285:dbl[])
        n2924 = Multiply(x=w4337, y=w4343) -> (x*y=w4344:dbl[])
        n2925 = Multiply(x=w4337, y=w4339) -> (x*y=w4340:dbl[])
        n2926 = Multiply(x=w4337, y=w4341) -> (x*y=w4342:dbl[])
        n2927 = Multiply(x=w4337, y=w4336) -> (x*y=w4338:dbl[])
        n2928 = Build Array (concatenate)(w4319, w4311) -> (w4321:dbl[])
        n2929 = Build Array (concatenate)(w4293, w4285) -> (w4295:dbl[])
        n2930 = Build Array (concatenate)(w4402, w4344) -> (w4411:dbl[])
        n2931 = Build Array (concatenate)(w4352, w4338) -> (w4406:dbl[])
        n2932 = Build Array (concatenate)(w4354, w4342) -> (w4410:dbl[])
        n2933 = Build Array (concatenate)(w4353, w4340) -> (w4409:dbl[])
        n2934 = Reshape Array(w4321, w4261, w4262) -> (w4317:dbl[][])
        n2935 = Reshape Array(w4295, w4261, w4262) -> (w4291:dbl[][])
        n2936 = Reshape Array(w4411, w4261, w4262) -> (w4389:dbl[][])
        n2937 = Reshape Array(w4406, w4261, w4262) -> (w4372:dbl[][])
        n2938 = Reshape Array(w4410, w4261, w4262) -> (w4364:dbl[][])
        n2939 = Reshape Array(w4409, w4261, w4262) -> (w4379:dbl[][])
        n2940 = Array Subset(array=w4317, index (col)=0 ("index"), length (col)=w4260) -> (w4316:dbl[][])  [unwired: 2 in]
        n2941 = Array Subset(array=w4317, index (col)=w4260) -> (w4314:dbl[][])  [unwired: 3 in]
        n2942 = Array Subset(array=w4291, index (col)=0 ("index"), length (col)=w4260) -> (w4290:dbl[][])  [unwired: 2 in]
        n2943 = Array Subset(array=w4291, index (col)=w4260) -> (w4288:dbl[][])  [unwired: 3 in]
        n2944 = Array Subset(array=w4379, index (col)=0 ("index"), length (col)=w4260) -> (w4384:dbl[][])  [unwired: 2 in]
        n2945 = Array Subset(array=w4379, index (col)=w4260) -> (w4382:dbl[][])  [unwired: 3 in]
        n2946 = Array Subset(array=w4389, index (col)=0 ("index"), length (col)=w4260) -> (w4388:dbl[][])  [unwired: 2 in]
        n2947 = Array Subset(array=w4389, index (col)=w4260) -> (w4386:dbl[][])  [unwired: 3 in]
        n2948 = Array Subset(array=w4364, index (col)=0 ("index"), length (col)=w4260) -> (w4370:dbl[][])  [unwired: 2 in]
        n2949 = Array Subset(array=w4364, index (col)=w4260) -> (w4368:dbl[][])  [unwired: 3 in]
        n2950 = Array Subset(array=w4372, index (col)=0 ("index"), length (col)=w4260) -> (w4377:dbl[][])  [unwired: 2 in]
        n2951 = Array Subset(array=w4372, index (col)=w4260) -> (w4375:dbl[][])  [unwired: 3 in]
        n2952 = for {
          tunnel: w4316 -> [w4421] mode=indexing
          tunnel: [w4420] -> w4315 mode=indexing
          workers-P: _ -> [_]
          n2953 = Reverse 1D Array(array=w4421) -> (reversed array=w4420:dbl[])
        }
        n2954 = for {
          tunnel: w4290 -> [w4419] mode=indexing
          tunnel: [w4418] -> w4289 mode=indexing
          workers-P: _ -> [_]
          n2955 = Reverse 1D Array(array=w4419) -> (reversed array=w4418:dbl[])
        }
        n2956 = for {
          tunnel: w4384 -> [w4427] mode=indexing
          tunnel: [w4426] -> w4383 mode=indexing
          workers-P: _ -> [_]
          n2957 = Reverse 1D Array(array=w4427) -> (reversed array=w4426:dbl[])
        }
        n2958 = for {
          tunnel: w4388 -> [w4429] mode=indexing
          tunnel: [w4428] -> w4387 mode=indexing
          workers-P: _ -> [_]
          n2959 = Reverse 1D Array(array=w4429) -> (reversed array=w4428:dbl[])
        }
        n2960 = for {
          tunnel: w4370 -> [w4423] mode=indexing
          tunnel: [w4422] -> w4369 mode=indexing
          workers-P: _ -> [_]
          n2961 = Reverse 1D Array(array=w4423) -> (reversed array=w4422:dbl[])
        }
        n2962 = for {
          tunnel: w4377 -> [w4425] mode=indexing
          tunnel: [w4424] -> w4376 mode=indexing
          workers-P: _ -> [_]
          n2963 = Reverse 1D Array(array=w4425) -> (reversed array=w4424:dbl[])
        }
        n2964 = Index Array(array=w4389, index (row)=0) -> (element=→"Waveform Graph":dbl[])  [unwired: 1 in]
        n2965 = Add(x=w4315, y=w4314) -> (x+y=w4301:dbl[][])
        n2966 = Add(x=w4289, y=w4288) -> (x+y=w4275:dbl[][])
        n2967 = Add(x=w4383, y=w4382) -> (x+y=w4381:dbl[][])
        n2968 = Add(x=w4387, y=w4386) -> (x+y=w4361:dbl[][])
        n2969 = Add(x=w4369, y=w4368) -> (x+y=w4367:dbl[][])
        n2970 = Add(x=w4376, y=w4375) -> (x+y=w4374:dbl[][])
        n2971 = Divide(x=w4367, y=2) -> (x/y=w4365:dbl[][])
        n2972 = Divide(x=w4381, y=2) -> (x/y=w4326:dbl[][])
        n2973 = To Single Precision Float(number=w4361) -> (single precision float=w4360:sgl[][])
        n2974 = To Single Precision Float(number=w4301) -> (single precision float=w4305:sgl[][])
        n2975 = To Single Precision Float(number=w4275) -> (single precision float=w4279:sgl[][])
        n2976 = Divide(x=w4374, y=2) -> (x/y=w4328:dbl[][])
        n2977 = Transpose 2D Array(2D array=w4365) -> (transposed array=→"Data map":dbl[][])
        n2978 = To Single Precision Float(number=w4326) -> (single precision float=w4332:sgl[][])
        n2979 = To Single Precision Float(number=w4328) -> (single precision float=w4329:sgl[][])
        n2980 = call "IMAQ ArrayToImage"("Image Pixels (Float)"=w4360, "Image"=w4298) -> ("Image Out"=w4363:T2)  [unwired: 8 in, 1 out]
        n2981 = call "IMAQ ArrayToImage"("Image Pixels (Float)"=w4305, "Image"=w4297) -> ("Image Out"=w4307:T2)  [unwired: 8 in, 1 out]
        n2982 = call "IMAQ ArrayToImage"("Image Pixels (Float)"=w4279, "Image"=w4271) -> ("Image Out"=w4281:T2)  [unwired: 8 in, 1 out]
        n2983 = call "IMAQ ArrayToImage"("Image Pixels (Float)"=w4332, "Image"=w4272) -> ("Image Out"=w4334:T2)  [unwired: 8 in, 1 out]
        n2984 = call "IMAQ Symmetry"("Type of Symmetry"=w4362, "Image Src"=w4363) -> ("Image Dst Out"=w4358:T2)  [unwired: 3 in, 1 out]
        n2985 = call "IMAQ ArrayToImage"("Image Pixels (Float)"=w4329, "Image"=w4273) -> ("Image Out"=w4331:T2)  [unwired: 8 in, 1 out]
        n2986 = call "IMAQ Symmetry"("Type of Symmetry"=w4306, "Image Src"=w4307) -> ("Image Dst Out"=w4303:T2)  [unwired: 3 in, 1 out]
        n2987 = call "IMAQ Symmetry"("Type of Symmetry"=w4280, "Image Src"=w4281) -> ("Image Dst Out"=w4277:T2)  [unwired: 3 in, 1 out]
        n2988 = call "IMAQ Symmetry"("Type of Symmetry"=w4333, "Image Src"=w4334) -> ("Image Dst Out"=→"Detection Laser X":T2)  [unwired: 3 in, 1 out]
        n2989 = call "IMAQ Symmetry"("Type of Symmetry"=w4330, "Image Src"=w4331) -> ("Image Dst Out"=→"Detection Laser Y":T2)  [unwired: 3 in, 1 out]
        n2990 = call "IMAQ Set Simple Calibration"("Calibration Axis Info"=T44 {"Origin Pixel"={"X"=0.0, "Y"=0.0}, "Angle Relative to Horizontal (deg)"=0.0, "Axis Reference"=0}, "Grid Descriptor"=T45 {"X Step"=0.3, "Y Step"=0.3, "Unit"=enum."Undefined"}, "Image"=w4358) -> ("Calibrated Image"=→"APD 1":T2)  [unwired: 7 in, 1 out]
        n2991 = call "IMAQ Set Simple Calibration"("Calibration Axis Info"=T44 {"Origin Pixel"={"X"=0.0, "Y"=0.0}, "Angle Relative to Horizontal (deg)"=0.0, "Axis Reference"=0}, "Grid Descriptor"=T45 {"X Step"=0.3, "Y Step"=0.3, "Unit"=enum."Undefined"}, "Image"=w4303) -> ("Calibrated Image"=→"APD 2":T2)  [unwired: 7 in, 1 out]
        n2992 = call "IMAQ Set Simple Calibration"("Calibration Axis Info"=T44 {"Origin Pixel"={"X"=0.0, "Y"=0.0}, "Angle Relative to Horizontal (deg)"=0.0, "Axis Reference"=0}, "Grid Descriptor"=T45 {"X Step"=0.3, "Y Step"=0.3, "Unit"=enum."Undefined"}, "Image"=w4277) -> ("Calibrated Image"=→"APD 3":T2)  [unwired: 7 in, 1 out]
      }
    }
    n2993 = case "For computing FFTs for display" shown="True" "Compute FFT" {
      tunnel: w3791 -> [_ w4901]
      frame False {
      }
      frame True {
        n2994 = Build Array("FFT 1 Choice 1", "FFT 1 Choice 2", "FFT 2 Choice 1", "FFT 2 Choice 2") -> (w4894:u16[])
        n2995 = Array Size(array=w4901) -> (size(s)=w4900:i32)
        n2996 = feedback-in #20(w4894) -> ()
        n2997 = feedback #20(u16[] [100, 100, 100, 100]) -> (w4895:u16[])
        n2998 = feedback-in #21("# Spectra to Ave.") -> ()
        n2999 = feedback #21("# Spectra to Ave.") -> (w4892:dbl)
        n3000 = Not Equal?(x="# Spectra to Ave.", y=w4892) -> (x != y?=w4891:bool)
        n3001 = Not Equal?(x=w4894, y=w4895) -> (x != y?=w4893:bool)
        n3002 = feedback #22(1.0) -> (w4878:dbl)
        n3003 = Compound Arithmetic op=OR("Reset FFT", w4893, w4891) -> (w4876:bool)
        n3004 = Select(t=1.0, s=w4876, f=w4878) -> (s? t:f=w4880:dbl)
        n3005 = Greater?(x=w4880, y="# Spectra to Ave.") -> (0:w4899:bool)
        n3006 = Increment(x=w4880) -> (x+1=w4879:dbl)
        n3007 = feedback-in #22(w4879) -> ()
        n3008 = local read "DMA Update Period (s)"() -> (w4874:dbl)
        n3009 = Multiply(x="# Spectra to Ave.", y=w4874) -> (x*y=→"Ave. Time (s)":dbl)
        n3010 = Build Array(cluster{"f0":dbl, "df":dbl, "magnitude":dbl[]} {"f0"=0.0, "df"=0.0, "magnitude"=[]} ("PSD")) -> (w4883:cluster{"f0":dbl, "df":dbl, "magnitude":dbl[]}[])
        n3011 = Build Array(w4883, w4883, w4883, w4883) -> (w4885:T54)
        n3012 = feedback #23(w4885) -> (w4890:T54)
        n3013 = for {
          N: 4 -> [_]
          tunnel: w4894 -> [w4923] mode=indexing
          tunnel: w4901 -> [w4924]
          tunnel: w4900 -> [w4926]
          tunnel: w4876 -> [w4919]
          tunnel: w4899 -> [w4918]
          tunnel: "# Spectra to Ave." -> [w4917]
          tunnel: [w4916] -> w4889 mode=indexing
          tunnel: w4890 -> [w4921] mode=indexing
          tunnel: [w4920] -> w4877 mode=indexing
          tunnel: w4880 -> [w4915]
          n3014 = Less?(x=w4923, y=w4926) -> (x < y?=w4925:bool)
          n3015 = Index Array(array=w4924, index=w4923) -> (element=w4922:waveform(dbl))
          n3016 = case shown="True" w4925 {
            tunnel: w4922 -> [_ w4943]
            tunnel: w4921 -> [w4928 w4941]
            tunnel: [w4928 w4929] -> w4920
            tunnel: w4919 -> [_ w4940]
            tunnel: w4918 -> [_ w4933]
            tunnel: w4917 -> [_ w4932]
            tunnel: [cluster{"f0":dbl, "df":dbl, "magnitude":dbl[]} {"f0"=0.0, "df"=0.0, "magnitude"=[]} ("PSD") w4934] -> w4916
            tunnel: w4915 -> [_ w4931]
            frame False {
            }
            frame True {
              n3017 = call <vilib>:"Std Deviation and Variance.vi"("X"=w4943) -> ("mean"=w4944:dbl)  [unwired: 1 in, 2 out]
              n3018 = Subtract(x=w4943, y=w4944) -> (x-y=w4942:waveform(dbl))
              n3019 = xnode "Spectral Measurements"("Signals"=w4942) -> ("PSD"=w4936:cluster{"f0":dbl, "df":dbl, "magnitude":dbl[]})  [unwired: 1 in, 1 out]
              n3020 = case shown="False" w4940 {
                tunnel: w4941 -> [w4953 _]
                tunnel: [w4949 w4958] -> w4929
                tunnel: w4936 -> [w4952 w4959]
                tunnel: w4933 -> [w4951 _]
                frame False {
                  n3021 = Build Array (concatenate)(w4953, w4952) -> (w4950:cluster{"f0":dbl, "df":dbl, "magnitude":dbl[]}[])
                  n3022 = case shown="True" w4951 {
                    tunnel: w4950 -> [w4954 w4957]
                    tunnel: [w4954 w4955] -> w4949
                    frame False {
                    }
                    frame True {
                      n3023 = Delete From Array(array=w4957, index=0) -> (array with subset deleted=w4955:cluster{"f0":dbl, "df":dbl, "magnitude":dbl[]}[])  [unwired: 1 in, 1 out]
                    }
                  }
                }
                frame True {
                  n3024 = Build Array(w4959) -> (w4958:cluster{"f0":dbl, "df":dbl, "magnitude":dbl[]}[])
                }
              }
              n3025 = for {
                tunnel: w4929 -> [w4948] mode=indexing
                tunnel: [w4947] -> w4939 mode=indexing
                workers-P: _ -> [_]
                n3026 = Unbundle By Name(w4948) -> ("magnitude"=w4947:dbl[])
              }
              n3027 = Transpose 2D Array(2D array=w4939) -> (transposed array=w4938:dbl[][])
              n3028 = for {
                tunnel: w4938 -> [w4946] mode=indexing
                tunnel: [w4945] -> w4937 mode=indexing
                workers-P: _ -> [_]
                n3029 = Add Array Elements(numeric array=w4946) -> (sum=w4945:dbl)
              }
              n3030 = Select(t=w4932, s=w4933, f=w4931) -> (s? t:f=w4930:dbl)
              n3031 = Divide(x=w4937, y=w4930) -> (x/y=w4935:dbl[])
              n3032 = Bundle By Name(cluster=w4936, "magnitude"=w4935) -> (w4934:cluster{"f0":dbl, "df":dbl, "magnitude":dbl[]})
            }
          }
        }
        n3033 = case shown="True" w4876 {
          tunnel: w4877 -> [w4908 w4914]
          tunnel: [w4908 w4909] -> w4875
          frame False {
          }
          frame True {
            n3034 = Array Subset(array=w4914, index (row)=0 ("index"), length (row)=4 ("length"), index (col)=0 ("index"), length (col)=1 ("length")) -> (w4909:T54)
          }
        }
        n3035 = feedback-in #23(w4875) -> ()
        n3036 = Split 1D Array(array=w4889, index=2) -> (first subarray=→"FFT 1":cluster{"f0":dbl, "df":dbl, "magnitude":dbl[]}[], second subarray=→"FFT 2":cluster{"f0":dbl, "df":dbl, "magnitude":dbl[]}[])
      }
    }
    n3037 = local read "T1 calibration"() -> (w3590:T6)
    n3038 = local read "T2 calibration"() -> (w3589:T5)
    n3039 = Unbundle By Name(w3579) -> ("Y"=w3588:dbl[])
    n3040 = Unbundle By Name(w3576) -> ("Y"=w3587:dbl[])
    n3041 = call "calibrate trap data.vi"("T2 cal"=w3589, "T2"=w3587, "T1 cal"=w3590, "T1"=w3588) -> ("T2 force (pN)"=w3580:dbl[], "T2 position (nm)"=w3581:dbl[], "T1 force (pN)"=w3582:dbl[], "T1 position (nm)"=w3583:dbl[])
    n3042 = Bundle By Name(cluster=w3579, "Y"=w3583) -> (w3578:waveform(dbl))
    n3043 = Bundle By Name(cluster=w3579, "Y"=w3582) -> (w3577:waveform(dbl))
    n3044 = Bundle By Name(cluster=w3576, "Y"=w3581) -> (w3575:waveform(dbl))
    n3045 = Bundle By Name(cluster=w3576, "Y"=w3580) -> (w3574:waveform(dbl))
    n3046 = Subtract(x=w3583, y=w3581) -> (x-y=w3835:dbl[])
    n3047 = case shown="True" "Read Lateness and Rel Phase" {
      tunnel: w3665 -> [w4205 w4238]
      tunnel: w3664 -> [w4206 w4237]
      tunnel: [w4205 w4210] -> w3833
      tunnel: [w4206 w4209] -> w3832
      frame False {
      }
      frame True {
        n3048 = xnode "Read/Write Control"("FPGA VI Reference In"=w4238, "error in"=w4237) -> ("FPGA VI Reference Out"=w4212:T24, "error out"=w4211:errorcluster, "GI Relative phase"=→"GI relative phase":i16, "Relative phase"=→"Relative phase (AI1)":i16, "AI Late Counter"=→"Late Counter (AI1)":u8, "GI Late Counter"=→"GI Late Counter":u8, "MCL Late Counter"=→"MCL Late Counter":u8, "MCL Relative Phase"=→"Relative Phase (MCL)":i16, "APD Acq Relative Phase"=→"APD Acq Relative Phase":i16, "APD 1 Gate Relative Phase"=→"APD 1 Gate Relative Phase":i16, "APD 2 Gate Relative Phase"=→"APD 2 Gate Relative Phase":i16, "APD Acq Late Counter"=→"APD Acq Late Counter":u8, "APD 1 Gate Late Counter"=→"APD 1 Gate Late Counter":u8, "APD 2 Gate Late Counter"=→"APD 2 Gate Late Counter":u8, "Green FB Relative Phase"=→"Relative phase (Green FB)":i16, "GI Relative phase 2"=→"GI relative phase 2":i16, "GI Late Counter 2"=→"GI Late Counter 2":u8, "Trap Pos FIFO Timeout"=→"Trap Pos FIFO Timeout":u16, "Trap AI FIFO Timeout"=→"Trap AI FIFO Timeout":u16, "RI Late Counter"=→"RI Late Counter":u8, "RI Relative phase"=→"RI relative phase":i16, "Green Late Counter"=→"Green AI Late Counter":u8, "BI Late Counter (AO)"=→"Late Counter (BI AO)":u8, "Blue Late Counter (D)"=→"Late Counter (BI DO)":u8, "BI Relative phase (AO)"=→"Relative phase (BI AO)":i16, "BI Relative phase (D)"=→"Relative phase (BI DO)":i16)
        n3049 = xnode "Read/Write Control"("FPGA VI Reference In"=w4212, "error in"=w4211) -> ("FPGA VI Reference Out"=w4210:T24, "error out"=w4209:errorcluster, "APD 3 Gate Late Counter"=→"APD 3 Gate Late Counter":u8, "APD 3 Gate Relative Phase"=→"APD 3 Gate Relative Phase":i16)